vi "Dresden R2R Sputter 03.02.2018 IY24.vi"() -> ()   [LabVIEW 2009] (continued)
                                }
                                frame #1 {
                                n29724 = local write "Ch4_WFC_do"(FALSE ("Ch1_WFC_do")) -> ()
                                n29725 = Wait Until Next ms Multiple(millisecond multiple=u32 200) -> ()  [unwired: 1 out]
                                }
                                }
                                n29726 = local read "Semi"() -> (w34638:bool)
                                n29727 = Or(x=w34639, y=w34638) -> (x .or. y?=w34637:bool)
                                }
                                }
                                frame #1 {
                                }
                                }
                                }
                                frame #1 {
                                n29728 = local read "Semi"() -> (w34650:bool)
                                n29729 = case shown="False" w34650 {
                                frame #0 {
                                n29730 = while {
                                i -> [w34656]
                                stop <- w34651 stop-if-true
                                n29731 = Greater?(x=w34656, y=100) -> (0:w34655:bool)
                                n29732 = case shown="True" w34655 {
                                frame #0 {
                                }
                                frame #1 {
                                n29733 = local write "Semi"(TRUE ("Semi")) -> ()
                                n29734 = local write "Error Message"("Coating Process  \nwas cancelled.\nPlease check water \nflow connection." ("Error Message")) -> ()
                                }
                                }
                                n29735 = local read "Ch1_WFS_di"() -> (w34654:bool)
                                n29736 = case shown="True" w34654 {
                                tunnel: [TRUE FALSE] -> w34653
                                frame #0 {
                                }
                                frame #1 {
                                n29737 = local write "Ch1_WFC_do"(FALSE ("Ch1_WFC_do")) -> ()
                                n29738 = Wait Until Next ms Multiple(millisecond multiple=u32 200) -> ()  [unwired: 1 out]
                                }
                                }
                                n29739 = local read "Semi"() -> (w34652:bool)
                                n29740 = Or(x=w34653, y=w34652) -> (x .or. y?=w34651:bool)
                                }
                                }
                                frame #1 {
                                }
                                }
                                }
                                frame #2 {
                                n29741 = local read "Semi"() -> (w34664:bool)
                                n29742 = case shown="False" w34664 {
                                frame #0 {
                                n29743 = while {
                                i -> [w34670]
                                stop <- w34665 stop-if-true
                                n29744 = Greater?(x=w34670, y=100) -> (0:w34669:bool)
                                n29745 = case shown="True" w34669 {
                                frame #0 {
                                }
                                frame #1 {
                                n29746 = local write "Semi"(TRUE ("Semi")) -> ()
                                n29747 = local write "Error Message"("Coating Process  \nwas cancelled.\nPlease check water \nflow connection." ("Error Message")) -> ()
                                }
                                }
                                n29748 = local read "Ch2_WFS_di"() -> (w34668:bool)
                                n29749 = case shown="True" w34668 {
                                tunnel: [TRUE FALSE] -> w34667
                                frame #0 {
                                }
                                frame #1 {
                                n29750 = local write "Ch2_WFC_do"(FALSE ("Ch1_WFC_do")) -> ()
                                n29751 = Wait Until Next ms Multiple(millisecond multiple=u32 200) -> ()  [unwired: 1 out]
                                }
                                }
                                n29752 = local read "Semi"() -> (w34666:bool)
                                n29753 = Or(x=w34667, y=w34666) -> (x .or. y?=w34665:bool)
                                }
                                }
                                frame #1 {
                                }
                                }
                                }
                                frame #3 {
                                n29754 = local read "Semi"() -> (w34678:bool)
                                n29755 = case shown="False" w34678 {
                                frame #0 {
                                n29756 = while {
                                i -> [w34684]
                                stop <- w34679 stop-if-true
                                n29757 = Greater?(x=w34684, y=100) -> (0:w34683:bool)
                                n29758 = case shown="True" w34683 {
                                frame #0 {
                                }
                                frame #1 {
                                n29759 = local write "Semi"(TRUE ("Semi")) -> ()
                                n29760 = local write "Error Message"("Coating Process  \nwas cancelled.\nPlease check water \nflow connection." ("Error Message")) -> ()
                                }
                                }
                                n29761 = local read "Ch3_WFS_di"() -> (w34682:bool)
                                n29762 = case shown="False" w34682 {
                                tunnel: [FALSE TRUE] -> w34681
                                frame #0 {
                                n29763 = local write "Ch3_WFC_do"(TRUE ("Ch1_WFC_do")) -> ()
                                n29764 = Wait Until Next ms Multiple(millisecond multiple=u32 200) -> ()  [unwired: 1 out]
                                }
                                frame #1 {
                                }
                                }
                                n29765 = local read "Semi"() -> (w34680:bool)
                                n29766 = Or(x=w34681, y=w34680) -> (x .or. y?=w34679:bool)
                                }
                                }
                                frame #1 {
                                }
                                }
                                }
                                frame #4 {
                                n29767 = local read "Semi"() -> (w34692:bool)
                                n29768 = case shown="False" w34692 {
                                frame #0 {
                                n29769 = local write "SDC1 2"(TRUE ("SDC1 2")) -> ()
                                n29770 = Wait (ms)(milliseconds to wait=u32 1000) -> ()  [unwired: 1 out]
                                }
                                frame #1 {
                                }
                                }
                                }
                                }
                                }
                                frame #2 {
                                # "BG-BV open"
                                n29771 = stacked-sequence {
                                frame #0 {
                                n29772 = local read "Semi"() -> (w34695:bool)
                                n29773 = case shown="False" w34695 {
                                frame #0 {
                                n29774 = while {
                                i -> [w34701]
                                stop <- w34696 stop-if-true
                                n29775 = Greater?(x=w34701, y=50) -> (0:w34700:bool)
                                n29776 = case shown="True" w34700 {
                                frame #0 {
                                }
                                frame #1 {
                                n29777 = local write "Semi"(TRUE ("Semi")) -> ()
                                n29778 = local write "Error Message"("Coating Process  \nwas cancelled.\nPlease check \nBG-BV connection." ("Error Message")) -> ()
                                }
                                }
                                n29779 = local read "Ch3_Bg_bv_di"() -> (w34699:bool)
                                n29780 = case shown="False" w34699 {
                                tunnel: [FALSE TRUE] -> w34698
                                frame #0 {
                                n29781 = local write "Ch3_Bg_bv_do"(TRUE ("Ch1_WFC_do")) -> ()
                                n29782 = Wait Until Next ms Multiple(millisecond multiple=u32 200) -> ()  [unwired: 1 out]
                                }
                                frame #1 {
                                }
                                }
                                n29783 = local read "Semi"() -> (w34697:bool)
                                n29784 = Or(x=w34698, y=w34697) -> (x .or. y?=w34696:bool)
                                }
                                }
                                frame #1 {
                                }
                                }
                                }
                                frame #1 {
                                n29785 = local read "Semi"() -> (w34709:bool)
                                n29786 = case shown="False" w34709 {
                                frame #0 {
                                n29787 = Wait (ms)(milliseconds to wait=u32 1000) -> ()  [unwired: 1 out]
                                n29788 = local write "SDC1 4"(TRUE ("SDC1 4")) -> ()
                                }
                                frame #1 {
                                }
                                }
                                }
                                }
                                }
                                frame #3 {
                                # "Baratron set zero"
                                n29789 = stacked-sequence {
                                frame #0 {
                                n29790 = local write "Pc_bv3_auto_baratron_set_zero"(TRUE ("Pc_bv2_auto_baratron_set_zero")) -> ()
                                }
                                frame #1 {
                                n29791 = while {
                                i -> [w34717]
                                stop <- w34714 stop-if-true
                                n29792 = Greater?(x=w34717, y=50 ("Baratron set zero time 2")) -> (0:w34716:bool)
                                n29793 = case shown="True" w34716 {
                                frame #0 {
                                }
                                frame #1 {
                                n29794 = local write "Semi"(TRUE ("Semi")) -> ()
                                n29795 = local write "Error Message"("" ("Error Message")) -> ()
                                }
                                }
                                n29796 = local read "Pressure_ch3"() -> (w34713:i32)
                                n29797 = Less?(x=w34713, y=0.1 ("Pressure Check for baratron set zero")) -> (x < y?=w34720:bool)
                                n29798 = case shown="False" w34720 {
                                tunnel: [FALSE TRUE] -> w34719
                                frame #0 {
                                n29799 = Wait Until Next ms Multiple(millisecond multiple=u32 200) -> ()  [unwired: 1 out]
                                }
                                frame #1 {
                                }
                                }
                                n29800 = local read "Semi"() -> (w34718:bool)
                                n29801 = Or(x=w34719, y=w34718) -> (x .or. y?=w34714:bool)
                                }
                                }
                                frame #2 {
                                n29802 = local read "Semi"() -> (w34727:bool)
                                n29803 = case shown="False" w34727 {
                                frame #0 {
                                n29804 = local write "SDC1 2b"(TRUE ("SDC1 2b")) -> ()
                                n29805 = Wait (ms)(milliseconds to wait=u32 1000) -> ()  [unwired: 1 out]
                                }
                                frame #1 {
                                }
                                }
                                }
                                }
                                }
                                frame #4 {
                                # "CC CLOSE"
                                n29806 = stacked-sequence {
                                frame #0 {
                                n29807 = local read "Semi"() -> (w34730:bool)
                                n29808 = case shown="False" w34730 {
                                frame #0 {
                                n29809 = while {
                                i -> [w34736]
                                stop <- w34731 stop-if-true
                                n29810 = Greater?(x=w34736, y=50) -> (0:w34735:bool)
                                n29811 = case shown="True" w34735 {
                                frame #0 {
                                }
                                frame #1 {
                                n29812 = local write "Semi"(TRUE ("Semi")) -> ()
                                n29813 = local write "Error Message"("Coating Process  \nwas cancelled.\nPlease check \nBG-BV connection." ("Error Message")) -> ()
                                }
                                }
                                n29814 = local read "Ch3_Cc_on_off_di"() -> (w34734:bool)
                                n29815 = case shown="True" w34734 {
                                tunnel: [TRUE FALSE] -> w34733
                                frame #0 {
                                }
                                frame #1 {
                                n29816 = local write "Ch3_Cc_on_off_do"(FALSE ("Ch1_WFC_do")) -> ()
                                n29817 = Wait Until Next ms Multiple(millisecond multiple=u32 200) -> ()  [unwired: 1 out]
                                }
                                }
                                n29818 = local read "Semi"() -> (w34732:bool)
                                n29819 = Or(x=w34733, y=w34732) -> (x .or. y?=w34731:bool)
                                }
                                }
                                frame #1 {
                                }
                                }
                                }
                                frame #1 {
                                n29820 = local read "Semi"() -> (w34744:bool)
                                n29821 = case shown="False" w34744 {
                                frame #0 {
                                n29822 = local write "SDC1 3"(TRUE ("SDC1 3")) -> ()
                                n29823 = Wait (ms)(milliseconds to wait=u32 1000) -> ()  [unwired: 1 out]
                                }
                                frame #1 {
                                }
                                }
                                }
                                }
                                }
                                frame #5 {
                                # "PC-BV CLOSE"
                                n29824 = stacked-sequence {
                                frame #0 {
                                n29825 = local read "Semi"() -> (w34747:bool)
                                n29826 = case shown="False" w34747 {
                                frame #0 {
                                n29827 = stacked-sequence {
                                frame #0 {
                                n29828 = local read "Semi"() -> (w34748:bool)
                                n29829 = case shown="False" w34748 {
                                frame #0 {
                                n29830 = local write "Pc_bv3_auto_close"(TRUE ("Tp1_auto_start")) -> ()
                                }
                                frame #1 {
                                }
                                }
                                }
                                frame #1 {
                                n29831 = local read "Semi"() -> (w34750:bool)
                                n29832 = case shown="False" w34750 {
                                frame #0 {
                                n29833 = Wait (ms)(milliseconds to wait=u32 1000) -> ()  [unwired: 1 out]
                                }
                                frame #1 {
                                }
                                }
                                }
                                frame #2 {
                                n29834 = local read "Semi"() -> (w34752:bool)
                                n29835 = case shown="False" w34752 {
                                frame #0 {
                                n29836 = while {
                                i -> [w34758]
                                stop <- w34754 stop-if-true
                                n29837 = local read "Pc_bv_closed_ch3"() -> (w34756:bool)
                                n29838 = Greater?(x=w34758, y=120) -> (0:w34757:bool)
                                n29839 = local read "Semi"() -> (w34755:bool)
                                n29840 = Compound Arithmetic op=OR(w34755, w34756, w34757) -> (w34754:bool)
                                n29841 = Wait (ms)(milliseconds to wait=u32 500) -> ()  [unwired: 1 out]
                                }
                                }
                                frame #1 {
                                }
                                }
                                }
                                frame #3 {
                                n29842 = local read "Semi"() -> (w34760:bool)
                                n29843 = case shown="False" w34760 {
                                frame #0 {
                                n29844 = local read "Pc_bv_closed_ch3"() -> (w34761:bool)
                                n29845 = case shown="False" w34761 {
                                frame #0 {
                                n29846 = local write "Pc_bv3_auto_close"(TRUE ("Pc_bv1_auto_open")) -> ()
                                }
                                frame #1 {
                                }
                                }
                                }
                                frame #1 {
                                }
                                }
                                }
                                frame #4 {
                                n29847 = local read "Semi"() -> (w34763:bool)
                                n29848 = case shown="False" w34763 {
                                frame #0 {
                                n29849 = local read "Pc_bv_closed_ch3"() -> (w34764:bool)
                                n29850 = case shown="False" w34764 {
                                frame #0 {
                                n29851 = Wait (ms)(milliseconds to wait=u32 1000) -> ()  [unwired: 1 out]
                                }
                                frame #1 {
                                }
                                }
                                }
                                frame #1 {
                                }
                                }
                                }
                                frame #5 {
                                n29852 = local read "Semi"() -> (w34766:bool)
                                n29853 = case shown="False" w34766 {
                                frame #0 {
                                n29854 = while {
                                i -> [w34772]
                                stop <- w34768 stop-if-true
                                n29855 = local read "Pc_bv_closed_ch3"() -> (w34770:bool)
                                n29856 = Greater?(x=w34772, y=120) -> (0:w34771:bool)
                                n29857 = local read "Semi"() -> (w34769:bool)
                                n29858 = Compound Arithmetic op=OR(w34769, w34770, w34771) -> (w34768:bool)
                                n29859 = Wait (ms)(milliseconds to wait=u32 500) -> ()  [unwired: 1 out]
                                }
                                }
                                frame #1 {
                                }
                                }
                                }
                                frame #6 {
                                n29860 = local read "Semi"() -> (w34774:bool)
                                n29861 = case shown="False" w34774 {
                                frame #0 {
                                n29862 = local read "Pc_bv_closed_ch3"() -> (w34775:bool)
                                n29863 = case shown="False" w34775 {
                                frame #0 {
                                n29864 = local write "Error Message"("Start up process  cancelled\nbecause  PC-BV not closed.\nPlease check PC-BV1 connections." ("Error Message")) -> ()
                                n29865 = Wait (ms)(milliseconds to wait=u32 1000) -> ()  [unwired: 1 out]
                                }
                                frame #1 {
                                }
                                }
                                }
                                frame #1 {
                                }
                                }
                                }
                                }
                                }
                                frame #1 {
                                }
                                }
                                }
                                frame #1 {
                                n29866 = local read "Semi"() -> (w34778:bool)
                                n29867 = case shown="False" w34778 {
                                frame #0 {
                                n29868 = local write "SDC1 5"(TRUE ("SDC1 5")) -> ()
                                n29869 = Wait (ms)(milliseconds to wait=u32 1000) -> ()  [unwired: 1 out]
                                }
                                frame #1 {
                                }
                                }
                                }
                                }
                                }
                                frame #6 {
                                # "SOV-AR OPEN"
                                n29870 = stacked-sequence {
                                frame #0 {
                                n29871 = local read "Semi"() -> (w34781:bool)
                                n29872 = case shown="False" w34781 {
                                frame #0 {
                                n29873 = while {
                                i -> [w34787]
                                stop <- w34782 stop-if-true
                                n29874 = Greater?(x=w34787, y=50) -> (0:w34786:bool)
                                n29875 = case shown="True" w34786 {
                                frame #0 {
                                }
                                frame #1 {
                                n29876 = local write "Semi"(TRUE ("Semi")) -> ()
                                n29877 = local write "Error Message"("Coating Process  \nwas cancelled.\nPlease check \nSOV-Ar connection." ("Error Message")) -> ()
                                }
                                }
                                n29878 = local read "Ch3_Sov_Ar_di"() -> (w34785:bool)
                                n29879 = case shown="False" w34785 {
                                tunnel: [FALSE TRUE] -> w34784
                                frame #0 {
                                n29880 = local write "Ch3_Sov_Ar_do"(TRUE ("Ch1_WFC_do")) -> ()
                                n29881 = Wait Until Next ms Multiple(millisecond multiple=u32 200) -> ()  [unwired: 1 out]
                                }
                                frame #1 {
                                }
                                }
                                n29882 = local read "Semi"() -> (w34783:bool)
                                n29883 = Or(x=w34784, y=w34783) -> (x .or. y?=w34782:bool)
                                }
                                }
                                frame #1 {
                                }
                                }
                                }
                                frame #1 {
                                n29884 = local read "Semi"() -> (w34795:bool)
                                n29885 = case shown="False" w34795 {
                                frame #0 {
                                n29886 = while {
                                i -> [w34800]
                                stop <- w34798 stop-if-true
                                n29887 = Greater?(x=w34800, y=5) -> (0:w34796:bool)
                                n29888 = Wait Until Next ms Multiple(millisecond multiple=u32 1000) -> ()  [unwired: 1 out]
                                n29889 = local read "Semi"() -> (w34799:bool)
                                n29890 = Or(x=w34796, y=w34799) -> (x .or. y?=w34798:bool)
                                }
                                }
                                frame #1 {
                                }
                                }
                                }
                                frame #2 {
                                n29891 = local read "Semi"() -> (w34802:bool)
                                n29892 = case shown="False" w34802 {
                                frame #0 {
                                n29893 = local write "SDC1 6"(TRUE ("SDC1 6")) -> ()
                                n29894 = Wait (ms)(milliseconds to wait=u32 1000) -> ()  [unwired: 1 out]
                                }
                                frame #1 {
                                }
                                }
                                }
                                }
                                }
                                frame #7 {
                                # "CHECK CHAMBER PRESSURE"
                                n29895 = stacked-sequence {
                                frame #0 {
                                n29896 = local read "Semi"() -> (w34805:bool)
                                n29897 = case shown="False" w34805 {
                                frame #0 {
                                n29898 = while {
                                i -> [w34813]
                                stop <- w34807 stop-if-true
                                n29899 = Greater?(x=w34813, y=300) -> (0:w34812:bool)
                                n29900 = case shown="True" w34812 {
                                frame #0 {
                                }
                                frame #1 {
                                n29901 = local write "Semi"(TRUE ("Semi")) -> ()
                                n29902 = local write "Error Message"("Coating Process cancelled.\nPlease check chamber \nconnections." ("Error Message")) -> ()
                                }
                                }
                                n29903 = local read "Ch_pg_press_ch3_gui"() -> (w34806:dbl)
                                n29904 = Greater Or Equal?(x=w34806, y=0.9 ("CHAMBER PRESSURE 4")) -> (x >= y?=w34810:bool)
                                n29905 = case shown="True" w34810 {
                                tunnel: [TRUE FALSE] -> w34809
                                frame #0 {
                                }
                                frame #1 {
                                n29906 = Wait Until Next ms Multiple(millisecond multiple=u32 200) -> ()  [unwired: 1 out]
                                }
                                }
                                n29907 = local read "Semi"() -> (w34808:bool)
                                n29908 = Or(x=w34809, y=w34808) -> (x .or. y?=w34807:bool)
                                }
                                }
                                frame #1 {
                                }
                                }
                                }
                                frame #1 {
                                n29909 = local read "Semi"() -> (w34820:bool)
                                n29910 = case shown="False" w34820 {
                                frame #0 {
                                n29911 = Wait (ms)(milliseconds to wait=u32 1000) -> ()  [unwired: 1 out]
                                n29912 = local write "SDC1 8"(TRUE ("SDC1 8")) -> ()
                                }
                                frame #1 {
                                }
                                }
                                }
                                }
                                }
                                frame #8 {
                                # "PC-BV OPEN"
                                n29913 = stacked-sequence {
                                frame #0 {
                                n29914 = local read "Semi"() -> (w34823:bool)
                                n29915 = case shown="False" w34823 {
                                frame #0 {
                                n29916 = stacked-sequence {
                                frame #0 {
                                n29917 = local read "Semi"() -> (w34824:bool)
                                n29918 = case shown="False" w34824 {
                                frame #0 {
                                n29919 = local write "Pc_bv3_auto_open"(TRUE ("Tp1_auto_start")) -> ()
                                }
                                frame #1 {
                                }
                                }
                                }
                                frame #1 {
                                n29920 = local read "Semi"() -> (w34826:bool)
                                n29921 = case shown="False" w34826 {
                                frame #0 {
                                n29922 = Wait (ms)(milliseconds to wait=u32 1000) -> ()  [unwired: 1 out]
                                }
                                frame #1 {
                                }
                                }
                                }
                                frame #2 {
                                n29923 = local read "Semi"() -> (w34828:bool)
                                n29924 = case shown="False" w34828 {
                                frame #0 {
                                n29925 = while {
                                i -> [w34834]
                                stop <- w34830 stop-if-true
                                n29926 = local read "Pc_bv_opened_ch3"() -> (w34832:bool)
                                n29927 = Greater?(x=w34834, y=120) -> (0:w34833:bool)
                                n29928 = local read "Semi"() -> (w34831:bool)
                                n29929 = Compound Arithmetic op=OR(w34831, w34832, w34833) -> (w34830:bool)
                                n29930 = Wait (ms)(milliseconds to wait=u32 500) -> ()  [unwired: 1 out]
                                }
                                }
                                frame #1 {
                                }
                                }
                                }
                                frame #3 {
                                n29931 = local read "Semi"() -> (w34836:bool)
                                n29932 = case shown="False" w34836 {
                                frame #0 {
                                n29933 = local read "Pc_bv_opened_ch3"() -> (w34837:bool)
                                n29934 = case shown="False" w34837 {
                                frame #0 {
                                n29935 = local write "Pc_bv3_auto_open"(TRUE ("Pc_bv1_auto_open")) -> ()
                                }
                                frame #1 {
                                }
                                }
                                }
                                frame #1 {
                                }
                                }
                                }
                                frame #4 {
                                n29936 = local read "Semi"() -> (w34839:bool)
                                n29937 = case shown="False" w34839 {
                                frame #0 {
                                n29938 = local read "Pc_bv_opened_ch3"() -> (w34840:bool)
                                n29939 = case shown="False" w34840 {
                                frame #0 {
                                n29940 = Wait (ms)(milliseconds to wait=u32 1000) -> ()  [unwired: 1 out]
                                }
                                frame #1 {
                                }
                                }
                                }
                                frame #1 {
                                }
                                }
                                }
                                frame #5 {
                                n29941 = local read "Semi"() -> (w34842:bool)
                                n29942 = case shown="False" w34842 {
                                frame #0 {
                                n29943 = while {
                                i -> [w34848]
                                stop <- w34844 stop-if-true
                                n29944 = local read "Pc_bv_opened_ch3"() -> (w34846:bool)
                                n29945 = Greater?(x=w34848, y=120) -> (0:w34847:bool)
                                n29946 = local read "Semi"() -> (w34845:bool)
                                n29947 = Compound Arithmetic op=OR(w34845, w34846, w34847) -> (w34844:bool)
                                n29948 = Wait (ms)(milliseconds to wait=u32 500) -> ()  [unwired: 1 out]
                                }
                                }
                                frame #1 {
                                }
                                }
                                }
                                frame #6 {
                                n29949 = local read "Semi"() -> (w34850:bool)
                                n29950 = case shown="False" w34850 {
                                frame #0 {
                                n29951 = local read "Pc_bv_opened_ch3"() -> (w34851:bool)
                                n29952 = case shown="False" w34851 {
                                frame #0 {
                                n29953 = local write "Error Message"("Start up process  cancelled\nbecause  PC-BV not opened.\nPlease check PC-BV1 connections." ("Error Message")) -> ()
                                n29954 = Wait (ms)(milliseconds to wait=u32 1000) -> ()  [unwired: 1 out]
                                }
                                frame #1 {
                                }
                                }
                                }
                                frame #1 {
                                }
                                }
                                }
                                }
                                }
                                frame #1 {
                                }
                                }
                                }
                                frame #1 {
                                n29955 = local read "Semi"() -> (w34854:bool)
                                n29956 = case shown="False" w34854 {
                                frame #0 {
                                n29957 = Wait (ms)(milliseconds to wait=u32 1000) -> ()  [unwired: 1 out]
                                n29958 = local write "SDC1 7"(TRUE ("SDC1 7")) -> ()
                                }
                                frame #1 {
                                }
                                }
                                }
                                }
                                }
                                frame #9 {
                                # "CC OPEN"
                                n29959 = stacked-sequence {
                                frame #0 {
                                n29960 = local read "Semi"() -> (w34857:bool)
                                n29961 = case shown="False" w34857 {
                                frame #0 {
                                n29962 = while {
                                i -> [w34863]
                                stop <- w34858 stop-if-true
                                n29963 = Greater?(x=w34863, y=50) -> (0:w34862:bool)
                                n29964 = case shown="True" w34862 {
                                frame #0 {
                                }
                                frame #1 {
                                n29965 = local write "Semi"(TRUE ("Semi")) -> ()
                                n29966 = local write "Error Message"("Coating Process  \nwas cancelled.\nPlease check \nBG-BV connection." ("Error Message")) -> ()
                                }
                                }
                                n29967 = local read "Ch3_Cc_on_off_di"() -> (w34861:bool)
                                n29968 = case shown="False" w34861 {
                                tunnel: [FALSE TRUE] -> w34860
                                frame #0 {
                                n29969 = local write "Ch3_Cc_on_off_do"(TRUE ("Ch1_WFC_do")) -> ()
                                n29970 = Wait Until Next ms Multiple(millisecond multiple=u32 200) -> ()  [unwired: 1 out]
                                }
                                frame #1 {
                                }
                                }
                                n29971 = local read "Semi"() -> (w34859:bool)
                                n29972 = Or(x=w34860, y=w34859) -> (x .or. y?=w34858:bool)
                                }
                                }
                                frame #1 {
                                }
                                }
                                }
                                frame #1 {
                                n29973 = local read "Semi"() -> (w34871:bool)
                                n29974 = case shown="False" w34871 {
                                frame #0 {
                                n29975 = while {
                                i -> [w34876]
                                stop <- w34874 stop-if-true
                                n29976 = Greater?(x=w34876, y=30) -> (0:w34872:bool)
                                n29977 = Wait Until Next ms Multiple(millisecond multiple=u32 1000) -> ()  [unwired: 1 out]
                                n29978 = local read "Semi"() -> (w34875:bool)
                                n29979 = Or(x=w34872, y=w34875) -> (x .or. y?=w34874:bool)
                                }
                                }
                                frame #1 {
                                }
                                }
                                }
                                frame #2 {
                                n29980 = local read "Semi"() -> (w34878:bool)
                                n29981 = case shown="False" w34878 {
                                frame #0 {
                                n29982 = Wait (ms)(milliseconds to wait=u32 1000) -> ()  [unwired: 1 out]
                                n29983 = local write "SDC1 7b"(TRUE ("SDC1 3")) -> ()
                                }
                                frame #1 {
                                }
                                }
                                }
                                }
                                }
                                frame #10 {
                                # "CHECK CHAMBER PRESSURE"
                                n29984 = stacked-sequence {
                                frame #0 {
                                n29985 = local read "Semi"() -> (w34881:bool)
                                n29986 = case shown="False" w34881 {
                                frame #0 {
                                n29987 = while {
                                i -> [w34889]
                                stop <- w34883 stop-if-true
                                n29988 = Greater?(x=w34889, y=300) -> (0:w34888:bool)
                                n29989 = case shown="True" w34888 {
                                frame #0 {
                                }
                                frame #1 {
                                n29990 = local write "Semi"(TRUE ("Semi")) -> ()
                                n29991 = local write "Error Message"("Coating Process cancelled.\nPlease check chamber \nconnections." ("Error Message")) -> ()
                                }
                                }
                                n29992 = local read "Ch_CC_press_ch3 2"() -> (w34882:dbl)
                                n29993 = Greater Or Equal?(x=w34882, y=5e-05 ("CHAMBER PRESSURE 5")) -> (x >= y?=w34886:bool)
                                n29994 = case shown="True" w34886 {
                                tunnel: [TRUE FALSE] -> w34885
                                frame #0 {
                                }
                                frame #1 {
                                n29995 = Wait Until Next ms Multiple(millisecond multiple=u32 200) -> ()  [unwired: 1 out]
                                }
                                }
                                n29996 = local read "Semi"() -> (w34884:bool)
                                n29997 = Or(x=w34885, y=w34884) -> (x .or. y?=w34883:bool)
                                }
                                }
                                frame #1 {
                                }
                                }
                                }
                                frame #1 {
                                n29998 = local read "Semi"() -> (w34896:bool)
                                n29999 = case shown="False" w34896 {
                                frame #0 {
                                n30000 = Wait (ms)(milliseconds to wait=u32 1000) -> ()  [unwired: 1 out]
                                n30001 = local write "SDC1 10"(TRUE ("SDC1 10")) -> ()
                                }
                                frame #1 {
                                }
                                }
                                }
                                }
                                }
                                frame #11 {
                                # "CC CLOSE"
                                n30002 = stacked-sequence {
                                frame #0 {
                                n30003 = local read "Semi"() -> (w34899:bool)
                                n30004 = case shown="False" w34899 {
                                frame #0 {
                                n30005 = while {
                                i -> [w34905]
                                stop <- w34900 stop-if-true
                                n30006 = Greater?(x=w34905, y=50) -> (0:w34904:bool)
                                n30007 = case shown="True" w34904 {
                                frame #0 {
                                }
                                frame #1 {
                                n30008 = local write "Semi"(TRUE ("Semi")) -> ()
                                n30009 = local write "Error Message"("Coating Process  \nwas cancelled.\nPlease check \nBG-BV connection." ("Error Message")) -> ()
                                }
                                }
                                n30010 = local read "Ch3_Cc_on_off_di"() -> (w34903:bool)
                                n30011 = case shown="True" w34903 {
                                tunnel: [TRUE FALSE] -> w34902
                                frame #0 {
                                }
                                frame #1 {
                                n30012 = local write "Ch3_Cc_on_off_do"(FALSE ("Ch1_WFC_do")) -> ()